vi "ContinousCameraStageV2.vi"() -> ()   [LabVIEW 2016] (continued)
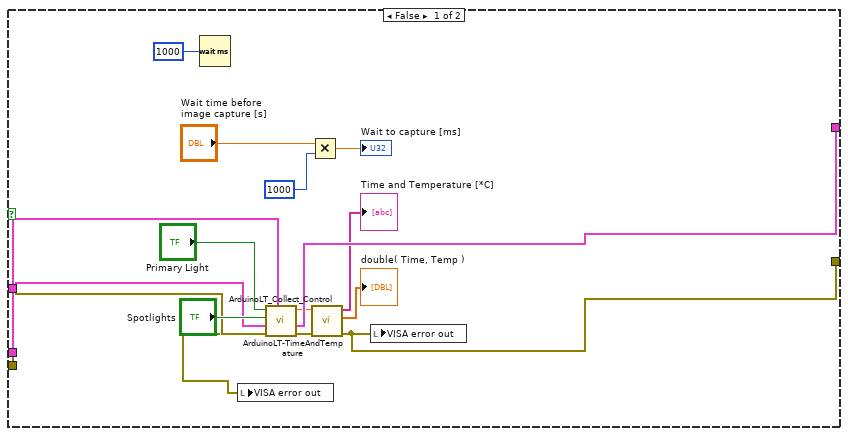
[diagram p2: hidden frame]
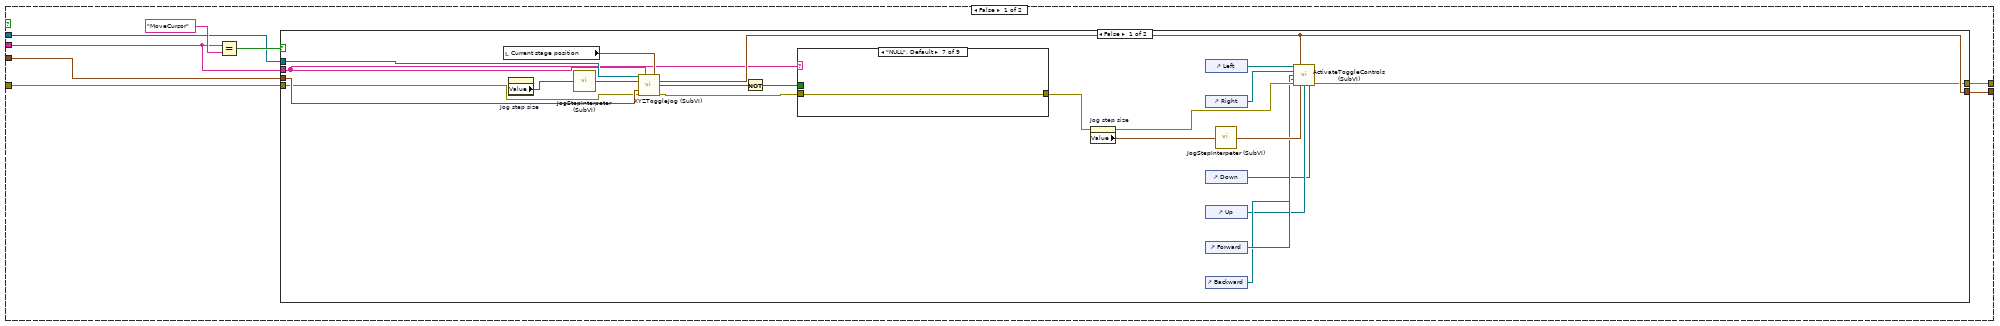
[diagram p4: hidden frame]
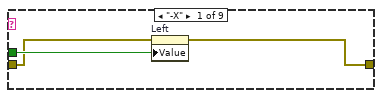
[diagram p5: hidden frame]
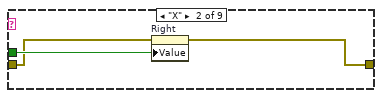
[diagram p6: hidden frame]
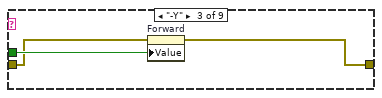
[diagram p7: hidden frame]
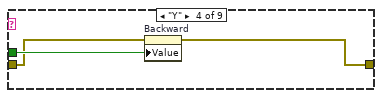
[diagram p8: hidden frame]
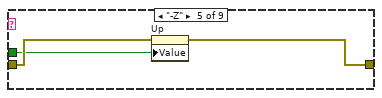
[diagram p9: hidden frame]
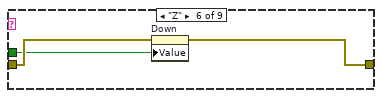
[diagram p10: hidden frame]
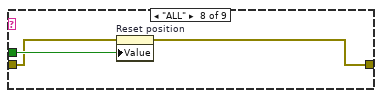
[diagram p11: hidden frame]
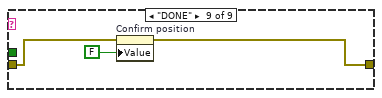
[diagram p12: hidden frame]
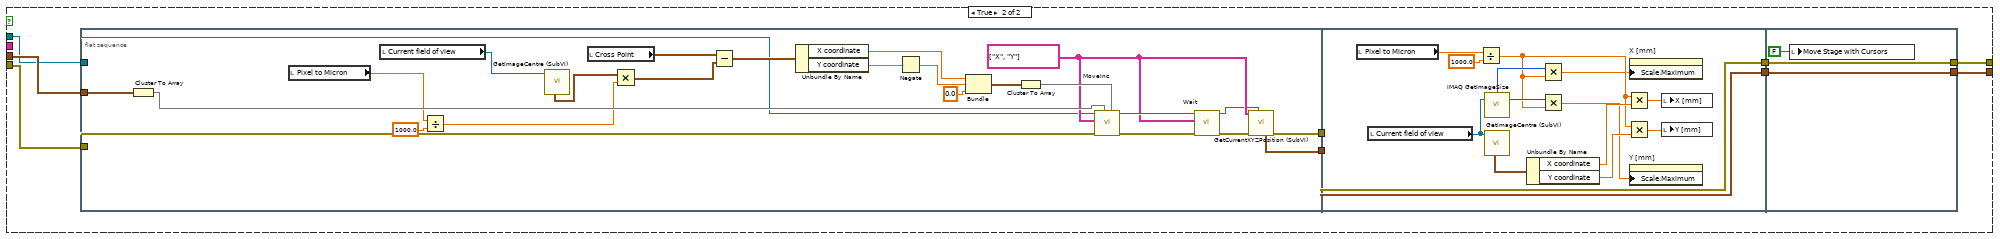
[diagram p13: hidden frame]
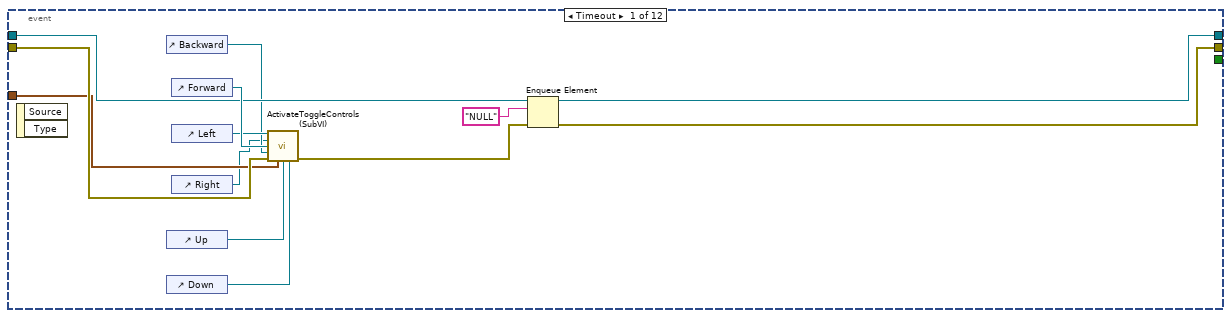
[diagram p14: hidden frame]
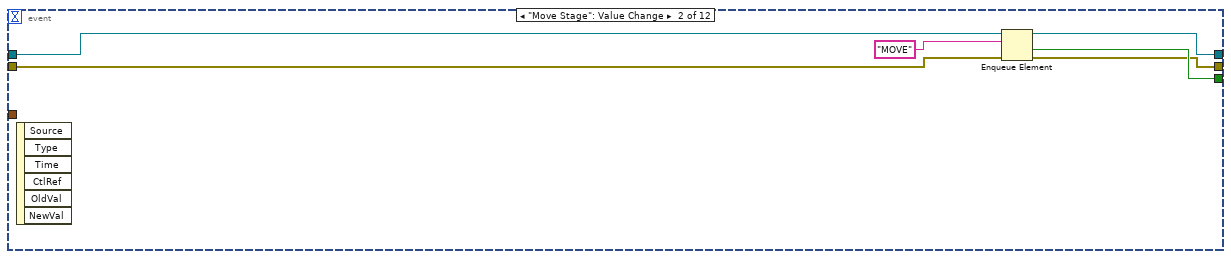
[diagram p15: hidden frame]
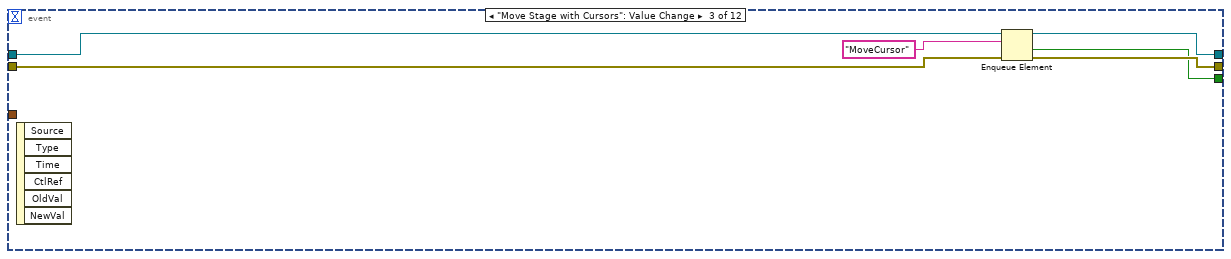
[diagram p16: hidden frame]
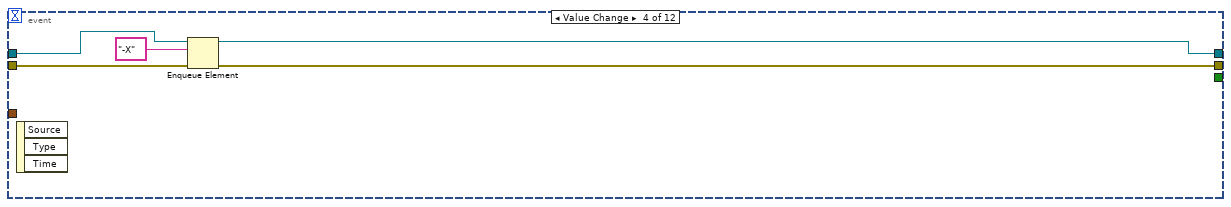
[diagram p17: hidden frame]
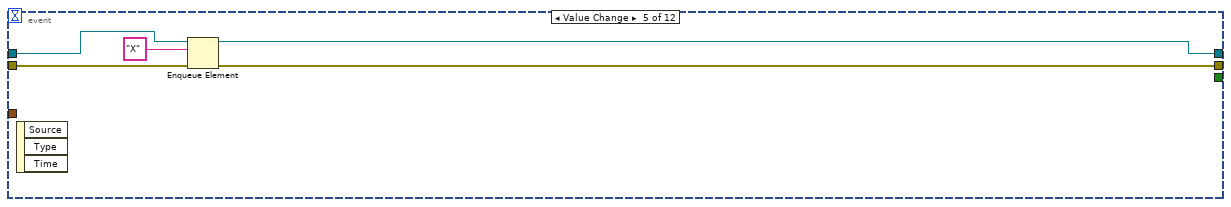
[diagram p18: hidden frame]
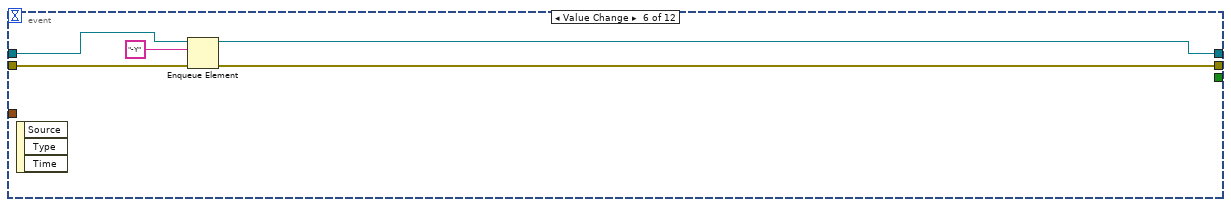
[diagram p19: hidden frame]
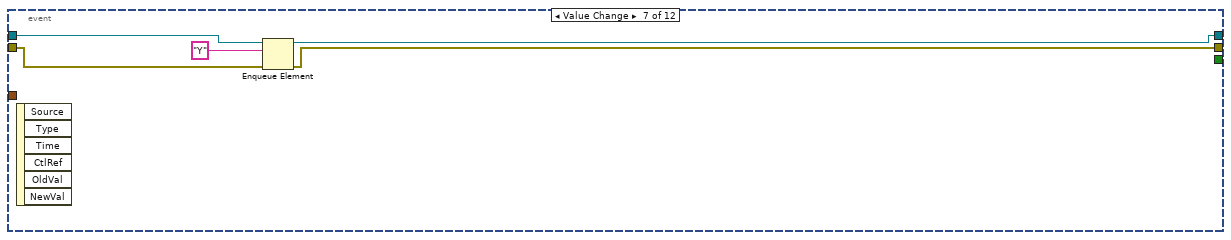
[diagram p20: hidden frame]
        n75 = disable-structure shown="Enabled" {
          disable-tunnel: [w248 w249] -> w244
          disable-tunnel: "Template Path" -> [w247 w249]
          frame Disabled {
            n76 = Build Path(base path=w247, name or relative path="Template") -> (appended path=w248:path)
          }
          frame Enabled {
          }
        }
        n77 = call "IMAQ Create"("Image Name"="untitled") -> ("New Image"=w239:T14, "error out"=w214:errorcluster)  [unwired: 4 in]
        n78 = call "IMAQ ReadFile"("File Path"=w244, "error in (no error)"=w214, "Image"=w239) -> ("error out"=w215:errorcluster, "Image Out"=w245:T14)  [unwired: 4 in, 3 out]
        "Template Image" <- w245
        n79 = call "IMAQ Find Pattern 4"("Image"=w240, "Template"=w245, "error in"=w215, "Settings"="Settings") -> ("Image Out"=w211:T14, "Matches (pixel)"=w237:T28)  [unwired: 5 in, 5 out]
        n80 = Array To Cluster(array=w237) -> (cluster=w236:T29)
        n81 = call "IMAQ GetImageSize"("Image"=w211) -> ("Y Resolution"=w225:i32, "X Resolution"=w228:i32)  [unwired: 3 in, 1 out]
        n82 = Unbundle By Name(w236) -> ("Matches (pixel)[0]"=w235:T30)
        n83 = Divide(x=w228, y=w227) -> (x/y=w216:dbl)
        n84 = Divide(x=w225, y=w227) -> (x/y=w226:dbl)
        n85 = local read "Pixel to Micron"() -> (w212:dbl)
        n86 = Unbundle By Name(w235) -> ("Position"=w238:cluster{"x":sgl, "y":sgl})
        n87 = local read "Current stage position"() -> (w242:T16)
        n88 = Unbundle By Name(w238) -> ("x"=w233:sgl, "y"=w234:sgl)
        n89 = Divide(x=w212, y=1000.0) -> (x/y=w231:dbl)
        n90 = Subtract(x=w233, y=w216) -> (x-y=w232:dbl)
        n91 = Subtract(x=w234, y=w226) -> (x-y=w210:dbl)
        n92 = Negate(x=w210) -> (-x=w209:dbl)
        n93 = Multiply(x=w232, y=w231) -> (x*y=w223:dbl)
        n94 = Multiply(x=w209, y=w231) -> (x*y=w222:dbl)
        n95 = Unbundle By Name(w242) -> ("X"=w224:dbl, "Y"=w221:dbl, "Z"=w218:dbl)
        n96 = Add(x=w223, y=w224) -> (x+y=w220:dbl)
        n97 = Add(x=w222, y=w221) -> (x+y=w219:dbl)
        n98 = Bundle(w223, w222) -> (→"1st Match Distance from Center":cluster{dbl, dbl})  [unwired: 1 in]
        n99 = Bundle(w220, w219, "Z"=w218) -> (→"1st Matched Position":cluster{dbl, dbl, "Z":dbl})  [unwired: 1 in]
      }
      frame "Analyze vignette" {
        n100 = call "Detect Brightness Maximum.vi"("Bullseye Color"=u32 6618880, "Threshold Max"="Threshold Max", "Refnum In"=w252) -> ("Eccentricity vs. Threshold"=→"Eccentricity vs. Threshold":cluster{i32[], dbl[]}, "Ellipses Out"=→"Ellipses Out":T14, "Bullseye Out"=w251:T14)  [unwired: 5 in, 1 out]
        "Bullseye Out" <- w251
      }
    }
    n101 = call <vilib>:"Simple Error Handler.vi"("error in (no error)"=w107) -> ("error out"=w104:errorcluster)  [unwired: 4 in, 4 out]
    n102 = call "IMAQ GetImageSize"("Image"=w86) -> ("Y Resolution"=w92:i32, "X Resolution"=w95:i32)  [unwired: 3 in, 1 out]
    n103 = call "IMAQ Histograph"("Image"=w86) -> ("Histogram Graph"=→"Intensity Histogram, current frame":T9)  [unwired: 7 in, 3 out]
    n104 = Compound Arithmetic op=OR(w105, w104) -> (w114:bool)
    n105 = Multiply(x=w93, y=w95) -> (x*y=w94:dbl)
    n106 = Multiply(x=w93, y=w92) -> (x*y=w91:dbl)
    n107 = property on="X [mm]" class="Slide (strict)"("Scale.Maximum"=w94) -> ()  [unwired: 2 in, 2 out]
    n108 = property on="Y [mm]" class="Slide (strict)"("Scale.Maximum"=w91) -> ()  [unwired: 2 in, 2 out]
    n109 = local read "Pixel to Micron"() -> (w88:dbl)
    n110 = call "DrawImageCentre (SubVI).vi"("Refnum in"=w87) -> ("Refnum out"=w103:T14)  [unwired: 9 in, 1 out]
    n111 = control-ref of="X [mm]"() -> (w100:refnum<vi>)
    n112 = control-ref of="Y [mm]"() -> (w101:refnum<vi>)
    n113 = call "UserSliderCursor (SubVI).vi"("Pixel to Micron"=w88, "Axes colour"=u32 2797823, "Coordinates Unit"=w89, "Image RefNum In"=w103, "Y slider refnum"=w101, "X slider refnum"=w100) -> ("Image Refnum out"=w102:T14, "Cross Point"=w90:cluster{"X coordinate":dbl, "Y coordinate":dbl})  [unwired: 3 in, 1 out]
    "Cross Point" <- w90
    n114 = Unbundle By Name(w90) -> ()  [unwired: 2 out]
    n115 = local write "Current field of view"(w102) -> ()
  }
  n116 = while "Producer Loop: Constantly collect camera image" {
    shift-right: [w269] -> w28
    shift-left: w21 -> [w270]
    shift-right: [w259] -> w27
    shift-left: w32 -> [w271]
    shift-right: [w261] -> w26
    shift-left: w29 -> [w264]
    stop <- w260 stop-if-true
    n117 = Unbundle By Name(w264) -> ("Camera session out"=w263:T8, "New Image"=w262:T14)
    n118 = call <vilib>:"IMAQdx Grab.vi"("error in"=w271, "Wait for Next Buffer? (Yes)"=TRUE, "Image In"=w262, "Session In"=w263) -> ("error out"=w268:errorcluster, "Image Out"=w256:T14, "Session Out"=w265:T8)  [unwired: 5 out]
    n119 = Bundle("Session Out"=w265, "Image Out"=w256) -> (w261:cluster{"Session Out":T8, "Image Out":T14})  [unwired: 1 in]
    n120 = Enqueue Element(queue=w270, element=w261, error in (no error)=w268) -> (queue out=w269:refnum<queue>, error out=w267:errorcluster)  [unwired: 1 in, 1 out]
    n121 = local read "Click to Stop The Program"() -> (w257:bool)
    n122 = call <vilib>:"Simple Error Handler.vi"("error in (no error)"=w267) -> ("error?"=w272:bool, "error out"=w259:errorcluster)  [unwired: 4 in, 3 out]
    "Camera error out" <- w259
    n123 = Unbundle By Name(w259) -> ("status"=w266:bool)
    n124 = Compound Arithmetic op=OR(w266, w257, w272) -> (w260:bool)
  }
  n125 = while "Cancel stage motion" {
    shift-right: [w274] -> _
    shift-left: w11 -> [w275]
    stop <- w273 stop-if-true
    n126 = case shown="True" "Abort stage" {
      tunnel: w275 -> [w277 w279]
      tunnel: [w277 w278] -> w274
      frame False {
      }
      frame True {
        n127 = call "AbortMultiple.vi"("axis names"=string[] ["X", "Y", "Z"], "controller in"=w279) -> ("controller out"=w278:refnum<k24>)  [unwired: 8 in, 1 out]
      }
    }
    n128 = local read "Click to Stop The Program"() -> (w273:bool)
  }
  n129 = while "Monitor XYZ stage axes: position, motion, homing, currents" {
    tunnel: w12 -> [w291]
    shift-right: [w288] -> _
    shift-left: w11 -> [w290]
    stop <- w281 stop-if-true
    n130 = Wait (ms)(milliseconds to wait=u32 100) -> ()  [unwired: 1 out]
    n131 = call "GetStageAxesStatus (SubVI).vi"(".NET Refnum in - Device"=w290, "Axes Names"=string[] ["X", "Y", "Z"], "error in (no error)"=w291) -> ("Homed"=→"Homed":bool, "Axis enabled"=→"Axis enabled":cluster{"X":bool, "Y ":bool, "Z":bool}, "Moving"=→"Moving":bool, ".NET Refnum out  - Device"=w288:refnum<k24>, "Current stage position"=→"Current stage position":T6, "Current monitoring"=→"Current monitoring":T31, "error out"=w287:errorcluster)  [unwired: 1 out]
    n132 = call <vilib>:"Simple Error Handler.vi"("error in (no error)"=w287) -> ("error out"=w292:errorcluster)  [unwired: 4 in, 4 out]
    n133 = local write "Program Errors 2"(w292) -> ()
    n134 = local read "Click to Stop The Program"() -> (w281:bool)
  }
  n135 = while "Consumer Loop: Interpret and execute jog instructions" {
    shift-right: [w296] -> _
    shift-left: w16 -> [w304]
    shift-right: [w297] -> _
    shift-left: w15 -> [w303]
    tunnel: w11 -> [w301]
    stop <- w298 stop-if-true
    n136 = Dequeue Element(queue=w304, error in (no error)=w303) -> (queue out=w296:refnum<queue>, element=w294:string, error out=w298:errorcluster)  [unwired: 1 in, 1 out]
    n137 = Equal?(x="MOVE" ("element"), y=w294) -> (x = y?=w302:bool)
    n138 = case shown="True" w302 {
      tunnel: w301 -> [w305 w418]
      tunnel: "Axes Speeds" -> [w310 w417]
      tunnel: [w307 w416] -> w299
      tunnel: w298 -> [w309 w415]
      tunnel: [w308 w414] -> w297
      tunnel: w294 -> [w306 _]
      frame False {
        n139 = Equal?(x=w306, y="MoveCursor") -> (x = y?=w311:bool)
        n140 = case shown="False" w311 {
          tunnel: [w325 w366] -> w307
          tunnel: w310 -> [w324 w368]
          tunnel: w309 -> [w323 w367]
          tunnel: w305 -> [w322 w364]
          tunnel: [w321 w365] -> w308
          tunnel: w306 -> [w319 _]
          frame False {
            n141 = local read "Current stage position"() -> (w320:T16)
            n142 = property on="Jog step size" class="Clust (strict)"() -> ("Value"=w331:T4)  [unwired: 2 in, 2 out]
            n143 = call "JogStepInterpeter (SubVI).vi"("Jog step size ENUM"=w331) -> ("Jog step size"=w330:T32)
            n144 = call "XYZToggleJog (SubVI).vi"("Aerotech in"=w322, "Motion direction"=w319, "Start location"=w320, "Jog step size"=w330, "Axis Speeds"=w324, "error in (no error)"=w323) -> ("Current stage position [mm]"=w325:cluster{"X":dbl, "Y":dbl, "Z":dbl}, "completed"=w326:bool, "error out"=w327:errorcluster)  [unwired: 5 in, 2 out]
            n145 = Not(x=w326) -> (.not. x?=w333:bool)
            n146 = case shown="\"NULL\", Default" w319 {
              tunnel: w333 -> [w336 w339 w343 w346 w348 w351 _ w356 _]
              tunnel: [w337 w340 w342 w345 w347 w350 w353 w355 w359] -> w328
              tunnel: w327 -> [w335 w338 w341 w344 w349 w352 w353 w354 w358]
              frame "-X" {
                n147 = property on="Left" class="Bool (strict)"(error in=w335, "Value"=w336) -> (error out=w337:errorcluster)  [unwired: 1 in, 1 out]
              }
              frame "X" {
                n148 = property on="Right" class="Bool (strict)"(error in=w338, "Value"=w339) -> (error out=w340:errorcluster)  [unwired: 1 in, 1 out]
              }
              frame "-Y" {
                n149 = property on="Forward" class="Bool (strict)"(error in=w341, "Value"=w343) -> (error out=w342:errorcluster)  [unwired: 1 in, 1 out]
              }
              frame "Y" {
                n150 = property on="Backward" class="Bool (strict)"(error in=w344, "Value"=w346) -> (error out=w345:errorcluster)  [unwired: 1 in, 1 out]
              }
              frame "-Z" {
                n151 = property on="Up" class="Bool (strict)"(error in=w349, "Value"=w348) -> (error out=w347:errorcluster)  [unwired: 1 in, 1 out]
              }
              frame "Z" {
                n152 = property on="Down" class="Bool (strict)"(error in=w352, "Value"=w351) -> (error out=w350:errorcluster)  [unwired: 1 in, 1 out]
              }
              frame "NULL", Default {
              }
              frame "ALL" {
                n153 = property on="Reset position" class="Bool (strict)"(error in=w354, "Value"=w356) -> (error out=w355:errorcluster)  [unwired: 1 in, 1 out]
              }
              frame "DONE" {
                n154 = property on="Confirm position" class="Bool (strict)"(error in=w358, "Value"=FALSE) -> (error out=w359:errorcluster)  [unwired: 1 in, 1 out]
              }
            }
            n155 = property on="Jog step size" class="Clust (strict)"(error in=w328) -> (error out=w329:errorcluster, "Value"=w318:T4)  [unwired: 1 in, 1 out]
            n156 = control-ref of="Left"() -> (w334:refnum<vi>)
            n157 = control-ref of="Right"() -> (w317:refnum<vi>)
            n158 = control-ref of="Down"() -> (w313:refnum<vi>)
            n159 = control-ref of="Up"() -> (w314:refnum<vi>)
            n160 = control-ref of="Forward"() -> (w316:refnum<vi>)
            n161 = control-ref of="Backward"() -> (w315:refnum<vi>)
            n162 = call "JogStepInterpeter (SubVI).vi"("Jog step size ENUM"=w318) -> ("Jog step size"=w332:T32)
            n163 = call "ActivateToggleControls (SubVI).vi"("Left refnum"=w334, "Current stage position [mm]"=w325, "Right refnum"=w317, "Forward refnum"=w316, "Backward refnum"=w315, "error in (no error)"=w329, "Jog step size"=w332, "Up refnum"=w314, "Down refnum"=w313) -> ("error out"=w321:errorcluster)  [unwired: 6 in]
          }
          frame True {
            n164 = flat-sequence {
              tunnel: w368 -> [w385]
              tunnel: w367 -> [w382]
              tunnel: w364 -> [w375]
              tunnel: [w380] -> w363
              tunnel: [w379] -> w361
              tunnel: w363 -> [w408]
              tunnel: [w408] -> w362
              tunnel: w361 -> [w407]
              tunnel: [w407] -> w360
              tunnel: [w410] -> w365
              tunnel: [w411] -> w366
              tunnel: w362 -> [w411]
              tunnel: w360 -> [w410]
              frame #0 {
                w378 = string[] ["X", "Y"] ("axis names")
                n165 = Cluster To Array(cluster=w385) -> (array=w384:dbl[])
                n166 = local read "Pixel to Micron"() -> (w373:dbl)
                n167 = local read "Current field of view"() -> (w376:T14)
                n168 = Divide(x=w373, y=1000.0) -> (x/y=w370:dbl)
                n169 = call "GetImageCentre (SubVI).vi"("Image in \n(refnum)"=w376) -> ("Centre Point"=w371:cluster{"X coordinate":dbl, "Y coordinate":dbl})  [unwired: 4 in, 4 out]
                n170 = local read "Cross Point"() -> (w374:cluster{"X coordinate":dbl, "Y coordinate":dbl})
                n171 = Multiply(x=w371, y=w370) -> (x*y=w369:cluster{"X coordinate":dbl, "Y coordinate":dbl})
                n172 = Subtract(x=w374, y=w369) -> (x-y=w392:cluster{"X coordinate":dbl, "Y coordinate":dbl})
                n173 = Unbundle By Name(w392) -> ("X coordinate"=w388:dbl, "Y coordinate"=w391:dbl)
                n174 = Negate(x=w391) -> (-x=w389:dbl)
                n175 = Bundle("X coordinate"=w388, w389, "y"=0.0) -> (w387:cluster{"X coordinate":dbl, dbl, "y":dbl})  [unwired: 1 in]
                n176 = Cluster To Array(cluster=w387) -> (array=w386:dbl[])
                n177 = call-poly "MoveInc.vi"("distances"=w386, "speeds"=w384, "error in (no error)"=w382, "axis names"=w378, "controller in"=w375) -> ("error out"=w381:errorcluster, "controller out"=w383:refnum<k24>)  [unwired: 5 in]
                n178 = call-poly "Wait.vi"("error in (no error)"=w381, "axis names"=w378, "controller in"=w383) -> ("error out"=w377:errorcluster, "controller out"=w372:refnum<k24>)  [unwired: 6 in, 1 out]
                n179 = call "GetCurrentXYZPosition (SubVI).vi"(".NET Refnum in - Device"=w372, "error in (no error)"=w377, "Axes Names"=w378) -> ("error out"=w379:errorcluster, "Current stage position"=w380:T6)  [unwired: 3 in, 4 out]
              }
              frame #1 {
                n180 = local read "Pixel to Micron"() -> (w400:dbl)
                n181 = local read "Current field of view"() -> (w406:T14)
                n182 = Divide(x=w400, y=1000.0) -> (x/y=w396:dbl)
                n183 = call "IMAQ GetImageSize"("Image"=w406) -> ("Y Resolution"=w397:i32, "X Resolution"=w398:i32)  [unwired: 3 in, 1 out]
                n184 = call "GetImageCentre (SubVI).vi"("Image in \n(refnum)"=w406) -> ("Centre Point"=w405:cluster{"X coordinate":dbl, "Y coordinate":dbl})  [unwired: 4 in, 4 out]
                n185 = Unbundle By Name(w405) -> ("X coordinate"=w401:dbl, "Y coordinate"=w402:dbl)
                n186 = Multiply(x=w398, y=w396) -> (x*y=w394:dbl)
                n187 = Multiply(x=w397, y=w396) -> (x*y=w395:dbl)
                n188 = Multiply(x=w396, y=w401) -> (x*y=w404:dbl)
                n189 = Multiply(x=w396, y=w402) -> (x*y=w403:dbl)
                n190 = property on="X [mm]" class="Slide (strict)"("Scale.Maximum"=w394) -> ()  [unwired: 2 in, 2 out]
                n191 = property on="Y [mm]" class="Slide (strict)"("Scale.Maximum"=w395) -> ()  [unwired: 2 in, 2 out]
                n192 = local write "X [mm]"(w404) -> ()
                n193 = local write "Y [mm]"(w403) -> ()
              }
              frame #2 {
                n194 = local write "Move Stage with Cursors"(FALSE) -> ()
              }
            }
          }
        }
      }
      frame True {
        n195 = flat-sequence {
          tunnel: w418 -> [w424]
          tunnel: w417 -> [w422]
          tunnel: w415 -> [w420]
          tunnel: [w421] -> w413
          tunnel: [w419] -> w412
          tunnel: [w426] -> w414
          tunnel: [w427] -> w416
          tunnel: w413 -> [w427]
          tunnel: w412 -> [w426]
          frame #0 {
            n196 = call "Go2XYZ (SubVI).vi"(".NET Refnum in"=w424, "Go to Coordinates"="Move to Absolute Position [mm]", "Axis Speeds"=w422, "error in (no error)"=w420) -> ("Final Position"=w421:T26, "error out"=w419:errorcluster)  [unwired: 7 in, 3 out]
          }
          frame #1 {
            n197 = local write "Move Stage"(FALSE) -> ()
          }
        }
      }
    }
    n198 = local write "Current stage position"(w299) -> ()
  }
  n199 = while "Producer Loop: Collect jog input instructions" {
    shift-right: [w441] -> w13
    shift-left: w15 -> [w432]
    shift-right: [w440] -> w14
    shift-left: w16 -> [w445]
    stop <- w443 stop-if-true
    n200 = Unbundle By Name("Jogging Controls") -> ("Jog step size"=w433:T4)
    n201 = local read "Current stage position"() -> (w430:T16)
    n202 = control-ref of="Left"() -> (w439:refnum<vi>)
    n203 = control-ref of="Right"() -> (w436:refnum<vi>)
    n204 = control-ref of="Up"() -> (w429:refnum<vi>)
    n205 = control-ref of="Backward"() -> (w438:refnum<vi>)
    n206 = control-ref of="Forward"() -> (w437:refnum<vi>)
    n207 = control-ref of="Down"() -> (w428:refnum<vi>)
    n208 = call "JogStepInterpeter (SubVI).vi"("Jog step size ENUM"=w433) -> ("Jog step size"=w431:T32)
    n209 = call "ActivateToggleControls (SubVI).vi"("Left refnum"=w439, "Current stage position [mm]"=w430, "Right refnum"=w438, "Forward refnum"=w437, "Backward refnum"=w436, "error in (no error)"=w432, "Jog step size"=w431, "Up refnum"=w429, "Down refnum"=w428) -> ("error out"=w435:errorcluster)  [unwired: 6 in]
    n210 = event shown="[9] \"Jogging Controls.Confirm position\": Value Change" {
      selector: _ -> [_ _ _ _ _ _ _ _ _ _ _ _]
      dyn-events: _ -> [_ _ _ _ _ _ _ _ _ _ _ _]
      timeout: _ -> [_ _ _ _ _ _ _ _ _ _ _ _]
      tunnel: w445 -> [w455 w464 w470 w474 w479 w485 w489 w494 w499 w506 w508 w516]
      tunnel: w435 -> [w454 w462 w468 w473 w478 w484 w488 w493 w498 w504 w509 w513]
      tunnel: [w452 w459 w466 w472 w477 w482 w487 w492 w497 w501 w510 w514] -> w441
      tunnel: [_ w460 w465 _ _ _ _ _ _ _ _ _] -> w442
      tunnel: [w451 w461 w467 w471 w476 w481 w486 w491 w496 w505 w511 w515] -> w440
      tunnel: w431 -> [w450 _ _ _ _ _ _ _ _ _ _ _]
      event Timeout {
        n211 = event-data() -> ()  [unwired: 1 in, 2 out]
        n212 = control-ref of="Backward"() -> (w449:refnum<vi>)
        n213 = control-ref of="Up"() -> (w447:refnum<vi>)
        n214 = control-ref of="Down"() -> (w446:refnum<vi>)
        n215 = control-ref of="Forward"() -> (w458:refnum<vi>)
        n216 = control-ref of="Left"() -> (w457:refnum<vi>)
        n217 = control-ref of="Right"() -> (w448:refnum<vi>)
        n218 = call "ActivateToggleControls (SubVI).vi"("Left refnum"=w457, "Right refnum"=w448, "Forward refnum"=w458, "Backward refnum"=w449, "error in (no error)"=w454, "Jog step size"=w450, "Up refnum"=w447, "Down refnum"=w446) -> ("error out"=w453:errorcluster)  [unwired: 7 in]
        n219 = Enqueue Element(queue=w455, element="NULL", error in (no error)=w453) -> (queue out=w451:refnum<queue>, error out=w452:errorcluster)  [unwired: 1 in, 1 out]
      }
      event "Move Stage": Value Change {
        n220 = event-data() -> ()  [unwired: 1 in, 6 out]
        n221 = Enqueue Element(queue=w464, element="MOVE", error in (no error)=w462) -> (queue out=w461:refnum<queue>, timed out?=w460:bool, error out=w459:errorcluster)  [unwired: 1 in]
      }
      event "Move Stage with Cursors": Value Change {
        n222 = event-data() -> ()  [unwired: 1 in, 6 out]
        n223 = Enqueue Element(queue=w470, element="MoveCursor", error in (no error)=w468) -> (queue out=w467:refnum<queue>, timed out?=w465:bool, error out=w466:errorcluster)  [unwired: 1 in]
      }
      event Value Change {
        n224 = event-data() -> ()  [unwired: 1 in, 3 out]
        n225 = Enqueue Element(queue=w474, element="-X", error in (no error)=w473) -> (queue out=w471:refnum<queue>, error out=w472:errorcluster)  [unwired: 1 in, 1 out]
      }
      event Value Change {
        n226 = event-data() -> ()  [unwired: 1 in, 3 out]
        n227 = Enqueue Element(queue=w479, element="X", error in (no error)=w478) -> (queue out=w476:refnum<queue>, error out=w477:errorcluster)  [unwired: 1 in, 1 out]
      }
      event Value Change {
        n228 = event-data() -> ()  [unwired: 1 in, 3 out]
        n229 = Enqueue Element(queue=w485, element="-Y", error in (no error)=w484) -> (queue out=w481:refnum<queue>, error out=w482:errorcluster)  [unwired: 1 in, 1 out]
      }
      event Value Change {
        n230 = event-data() -> ()  [unwired: 1 in, 6 out]
        n231 = Enqueue Element(queue=w489, element="Y", error in (no error)=w488) -> (queue out=w486:refnum<queue>, error out=w487:errorcluster)  [unwired: 1 in, 1 out]
      }
      event Value Change {
        n232 = event-data() -> ()  [unwired: 1 in, 3 out]
        n233 = Enqueue Element(queue=w494, element="-Z", error in (no error)=w493) -> (queue out=w491:refnum<queue>, error out=w492:errorcluster)  [unwired: 1 in, 1 out]
      }
      event Value Change {
        n234 = event-data() -> ()  [unwired: 1 in, 3 out]
        n235 = Enqueue Element(queue=w499, element="Z", error in (no error)=w498) -> (queue out=w496:refnum<queue>, error out=w497:errorcluster)  [unwired: 1 in, 1 out]
      }
      event Value Change {
        n236 = event-data() -> ()  [unwired: 1 in, 6 out]
        n237 = Enqueue Element(queue=w506, element="DONE", error in (no error)=w504) -> (queue out=w505:refnum<queue>, error out=w502:errorcluster)  [unwired: 1 in, 1 out]
        n238 = property on="Confirm position" class="Bool (strict)"(error in=w502, "Value"=FALSE ("Confirm position")) -> (error out=w501:errorcluster)  [unwired: 1 in, 1 out]
      }
      event Value Change {
        n239 = event-data() -> ()  [unwired: 1 in, 6 out]
        n240 = Enqueue Element(queue=w508, element="ALL", error in (no error)=w509) -> (queue out=w511:refnum<queue>, error out=w510:errorcluster)  [unwired: 1 in, 1 out]
      }
      event "Save current position": Value Change {
        n241 = event-data() -> ()  [unwired: 1 in, 5 out]
        n242 = local write "Save current position"(FALSE ("Save current position")) -> ()
        n243 = Enqueue Element(queue=w516, element="NULL", error in (no error)=w513) -> (queue out=w515:refnum<queue>, error out=w514:errorcluster)  [unwired: 1 in, 1 out]
        n244 = local read "Current stage position"() -> (w519:T16)
        n245 = local write "Move to Absolute Position [mm]"(w519) -> ()
      }
    }
    n246 = Unbundle By Name(w441) -> ("status"=w444:bool)
    n247 = Or(x=w444, y=w442) -> (x .or. y?=w443:bool)
  }
  n248 = call <vilib>:"Close.vi"("Arduino Resource"=w6, "error in"=w4) -> ("error out"=w5:errorcluster)  [unwired: 13 in]
  n249 = local write "VISA error out"(w5) -> ()
  n250 = Release Queue(queue=w28, error in (no error)=w27) -> (error out=w22:errorcluster)  [unwired: 1 in, 2 out]
  n251 = Unbundle(w26) -> ("Camera session out"=w25:T8, "New Image"=w24:T14)
  n252 = call "IMAQ Dispose"("Image"=w24, "error in (no error)"=w22) -> ("error out"=w23:errorcluster)  [unwired: 4 in]
  n253 = call <vilib>:"IMAQdx Close Camera.vi"("error in"=w23, "Session In"=w25) -> ("error out"=w20:errorcluster)  [unwired: 9 in]
  n254 = local write "Camera error out"(w20) -> ()
  n255 = Release Queue(queue=w14, error in (no error)=w13) -> ()  [unwired: 1 in, 3 out]
